vi "UHR-Fleezers Control (host) - Avogadro v2.vi"() -> ()   [LabVIEW 2014] (continued)
            n469 = local write "Stage Control Serial Error"(w819) -> ()
            n470 = Unbundle(w816) -> (w823:dbl, w825:dbl, w821:dbl)
            n471 = Add(x=w825, y="Y change (mm)") -> (x+y=w822:dbl)
            n472 = Bundle(w823, w822, w821) -> (w820:cluster{dbl, dbl, dbl})  [unwired: 1 in]
          }
          frame #1 {
            # "move to new position and start saving"
            n473 = local write "Stage Moving"(TRUE ("Stage Moving")) -> ()
            n474 = local write "Start Saving"(TRUE ("Start Saving")) -> ()
            n475 = call "Set Stage Position.vi"("Position"=w833, "error in"=w832, "VISA resource name in"=w831) -> ("error out"=w829:errorcluster, "VISA resource name out"=w830:refnum<visa-resource-name>)  [unwired: 1 out]
          }
          frame #2 {
            # "go back to start"
            n476 = call "Set Stage Position.vi"("Position"=w835, "error in"=w836, "VISA resource name in"=w837) -> ()  [unwired: 3 out]
          }
          frame #3 {
            # "stop saving"
            n477 = local write "Stop Saving"(TRUE ("Stop Saving")) -> ()
            n478 = local write "Stage Moving"(FALSE ("Stage Moving")) -> ()
          }
        }
      }
      event "Move to Position 1", "Move to Position 2", "Move to Position 3", "Move to Position 4", "Move to Position 5", "Lower Ch. Cap.", "Move to Position 6": Value Change {
        w840 = FALSE
        n479 = event-data() -> ()  [unwired: 1 in, 5 out]
        n480 = Or(x="Move to Position 5", y="Lower Ch. Cap.") -> (x .or. y?=w845:bool)
        n481 = Build Array("Move to Position 1", "Move to Position 2", "Move to Position 3", "Move to Position 4", w845, "Move to Position 6") -> (w848:bool[])
        n482 = local write "Move to Position 1"(w840) -> ()
        n483 = local write "Move to Position 2"(w840) -> ()
        n484 = local write "Move to Position 3"(w840) -> ()
        n485 = local write "Move to Position 4"(w840) -> ()
        n486 = local write "Move to Position 5"(w840) -> ()
        n487 = local write "Move to Position 6"(w840) -> ()
        n488 = Boolean Array To Number(Boolean array=w848) -> (number=w847:u32)
        n489 = Logarithm Base 2(1:w847) -> (0:w846:dbl)
        n490 = flat-sequence {
          tunnel: w846 -> [w857]
          tunnel: w843 -> [w855]
          tunnel: w842 -> [w854]
          frame #0 {
            n491 = local read "Saved Stage Positions"() -> (w865:dbl[][])
            n492 = Array Subset(array=w865, index (row)=w857, length (row)=1 ("length"), index (col)=1 ("index"), length (col)=3 ("length")) -> (w862:dbl[][])
            n493 = Reshape Array(w862, 3 ("dimension size")) -> (w860:dbl[])
            n494 = Array To Cluster(array=w860) -> (cluster=w859:cluster{"[0]":dbl, "[1]":dbl, "[2]":dbl})
            n495 = call "Set Stage Position.vi"("Position"=w859, "error in"=w854, "VISA resource name in"=w855) -> ("error out"=w858:errorcluster)  [unwired: 2 out]
            n496 = local write "Stage Moving"(TRUE ("Stage Moving")) -> ()
            n497 = local write "Stage Control Serial Error"(w858) -> ()
          }
          frame #1 {
            n498 = local write "Stage Moving"(FALSE ("Stage Moving")) -> ()
            n499 = call <vilib>:"Beep.vi"() -> ()  [unwired: 3 in, 9 out]
          }
        }
      }
      event "Force FB Data\nScript": Value Change {
        n500 = event-data() -> ()  [unwired: 1 in, 5 out]
        n501 = flat-sequence {
          tunnel: w873 -> [w877]
          tunnel: w874 -> [w878]
          tunnel: [w878] -> w869
          tunnel: [w877] -> w868
          tunnel: w869 -> [w881]
          tunnel: w868 -> [w880]
          tunnel: ["Trap Trig Fl."] -> w870
          tunnel: [w906] -> w871
          tunnel: w870 -> [w906]
          tunnel: [w910] -> w872
          tunnel: w871 -> [w910]
          tunnel: w872 -> [w912]
          frame #0 {
            n502 = property on="Trap Delta (MHz)" class="DigNum (strict)"("Val(Sgnl)"="Trap Delta Before Moving") -> ()  [unwired: 2 in, 2 out]
          }
          frame #1 {
            n503 = local read "Saved Stage Positions"() -> (w883:dbl[][])
            n504 = property on="Trap Pos. FB Offset Factor" class="DigNum (strict)"("Val(Sgnl)"=i64 0 ("Value (Signaling)")) -> ()  [unwired: 2 in, 2 out]
            n505 = local write "FB Trap Pos Offset"(0.0 ("FB Trap Pos Offset")) -> ()
            n506 = local write "Stage Moving"(TRUE ("Stage Moving")) -> ()
            n507 = call "move to saved stage position.vi"("error in"=w880, "Stage VISA resource name in"=w881, "Position"="Stage Position To Establish FB", "Saved Stage Positions"=w883) -> ("error out"=w879:errorcluster)  [unwired: 1 out]
            n508 = local write "Stage Control Serial Error"(w879) -> ()
          }
          frame #2 {
            n509 = call <vilib>:"Beep.vi"() -> ()  [unwired: 3 in, 9 out]
            n510 = Multiply(x="Wait (s)", y=u32 1000 ("milliseconds to wait")) -> (x*y=w890:u32)
            n511 = property on="Trap Delta (MHz)" class="DigNum (strict)"("Val(Sgnl)"="Starting \nTrap Delta (MHz)") -> ()  [unwired: 2 in, 2 out]
            n512 = local write "Stage Moving"(FALSE ("Stage Moving")) -> ()
            n513 = Wait (ms)(milliseconds to wait=w890) -> ()  [unwired: 1 out]
            n514 = property on="Tab Control 2" class="TabCtl (strict)"("Val(Sgnl)"=T15."Feedback on Trap Position" ("Value (Signaling)")) -> ()  [unwired: 2 in, 2 out]
            n515 = property on="Tab Control" class="TabCtl (strict)"("Val(Sgnl)"=T47."Trap Control (RF)" ("Value (Signaling)")) -> ()  [unwired: 2 in, 2 out]
          }
          frame #3 {
            n516 = property on="Set Reading to\nSetpoint" class="Bool (strict)"("Val(Sgnl)"=TRUE ("Value (Signaling)")) -> ()  [unwired: 2 in, 2 out]
            n517 = Wait (ms)(milliseconds to wait=u32 500) -> ()  [unwired: 1 out]
          }
          frame #4 {
            n518 = property on="Trap Pos. FB ON" class="Bool (strict)"("Val(Sgnl)"=TRUE ("Value (Signaling)")) -> ()  [unwired: 2 in, 2 out]
            n519 = Wait (ms)(milliseconds to wait=u32 250) -> ()  [unwired: 1 out]
          }
          frame #5 {
            n520 = case shown="False" "Trap Trig Fl." {
              frame False {
                n521 = case shown="True" "Green ON after FB ON?" {
                  selector: "Green ON after FB ON?" -> [_ w905]
                  frame False {
                  }
                  frame True {
                    n522 = property on="Green Laser ON" class="Bool (strict)"("Val(Sgnl)"=w905) -> ()  [unwired: 2 in, 2 out]
                  }
                }
              }
              frame True {
              }
            }
            n523 = case shown="True" "Remove Action Offset" {
              tunnel: TRUE ("Value (Signaling)") -> [w902 w903]
              frame False {
                n524 = property on="Remove Unwinding Offset" class="Bool (strict)"("Val(Sgnl)"=w902) -> ()  [unwired: 2 in, 2 out]
              }
              frame True {
                n525 = property on="Remove Action Offset" class="Bool (strict)"("Val(Sgnl)"=w903) -> ()  [unwired: 2 in, 2 out]
              }
            }
            n526 = Wait (ms)(milliseconds to wait=u32 250) -> ()  [unwired: 1 out]
          }
          frame #6 {
            n527 = property on="Start Saving" class="Bool (strict)"("Val(Sgnl)"=TRUE ("Value (Signaling)")) -> ()  [unwired: 2 in, 2 out]
            n528 = Wait (ms)(milliseconds to wait=u32 5000) -> ()  [unwired: 1 out]
          }
          frame #7 {
            w909 = TRUE ("Value (Signaling)")
            n529 = property on="Rem fb disp offset" class="Bool (strict)"("Val(Sgnl)"=w909) -> ()  [unwired: 2 in, 2 out]
            n530 = property on="Remove Offset" class="Bool (strict)"("Val(Sgnl)"=w909) -> ()  [unwired: 2 in, 2 out]
            n531 = Wait (ms)(milliseconds to wait=u32 100) -> ()  [unwired: 1 out]
          }
          frame #8 {
            n532 = case shown="True" w912 {
              frame False {
              }
              frame True {
                n533 = local write "Trap Trig. Fl."(TRUE ("Value (Signaling)")) -> ()
              }
            }
          }
          frame #9 {
            n534 = case shown="True" "Start dipping after?" {
              frame False {
              }
              frame True {
                n535 = flat-sequence {
                  frame #0 {
                    n536 = Multiply(x="Delay before dipping (s)", y=1000.0) -> (x*y=w916:dbl)
                    n537 = Wait (ms)(milliseconds to wait=w916) -> ()  [unwired: 1 out]
                  }
                  frame #1 {
                    n538 = property on="Dip for Protein" class="Bool (strict)"("Val(Sgnl)"=TRUE ("Value (Signaling)")) -> ()  [unwired: 2 in, 2 out]
                    n539 = local write "Scripts"(T3."Dipping" ("Scripts")) -> ()
                  }
                }
              }
            }
          }
        }
      }
      event "Fixed Traps Data\nScript": Value Change {
        n540 = event-data() -> ()  [unwired: 1 in, 5 out]
        n541 = flat-sequence {
          frame #0 {
            n542 = case shown="True" "Green ON" {
              frame False {
              }
              frame True {
                n543 = property on="Green Laser ON" class="Bool (strict)"("Val(Sgnl)"=TRUE) -> ()  [unwired: 2 in, 2 out]
              }
            }
            n544 = local write "Offset (nm)"(0.0 ("Offset (nm)")) -> ()
            n545 = property on="Sample Channel\nFlow" class="Bool (strict)"("Val(Sgnl)"=FALSE ("Value (Signaling)")) -> ()  [unwired: 2 in, 2 out]
            n546 = property on="Trap Delta (MHz)" class="DigNum (strict)"("Val(Sgnl)"="Fixed Traps Trap Delta (MHz)") -> ()  [unwired: 2 in, 2 out]
          }
          frame #1 {
            n547 = Wait (ms)(milliseconds to wait=u32 1000) -> ()  [unwired: 1 out]
          }
          frame #2 {
            n548 = local write "Start Saving"(TRUE ("Start Saving")) -> ()
          }
          frame #3 {
            n549 = local read "Bead Sep. Int. Time (s)"() -> (w927:dbl)
            n550 = Multiply(x=w927, y=1000.0) -> (x*y=w929:dbl)
            n551 = Wait (ms)(milliseconds to wait=w929) -> ()  [unwired: 1 out]
          }
          frame #4 {
            n552 = property on="Remove Offset" class="Bool (strict)"("Val(Sgnl)"=TRUE ("Value (Signaling)")) -> ()  [unwired: 2 in, 2 out]
          }
          frame #5 {
            n553 = property on="Dip for Protein" class="Bool (strict)"("Val(Sgnl)"="Start dipping after?") -> ()  [unwired: 2 in, 2 out]
          }
        }
      }
      event "Experiment position", "Get Bead 1", "Get bead 2", "Get bead 3": Value Change {
        w932 = FALSE
        n554 = event-data() -> ()  [unwired: 1 in, 6 out]
        n555 = Build Array("Get Bead 1", "Get bead 2", "Get bead 3", "Experiment position") -> (w937:bool[])
        n556 = Boolean Array To Number(Boolean array=w937) -> (number=w936:u32)
        n557 = local write "Get bead 3"(w932) -> ()
        n558 = local write "Get Bead 1"(w932) -> ()
        n559 = local write "Experiment position"(w932) -> ()
        n560 = local write "Get bead 2"(w932) -> ()
        n561 = Logarithm Base 2(1:w936) -> (0:w935:dbl)
        n562 = To Unsigned Long Integer(number=w935) -> (unsigned 32bit integer=w934:u32)
        n563 = case shown="3" w934 {
          frame 0, Default {
            n564 = property on="Move to Position 1" class="Bool (strict)"("Val(Sgnl)"=TRUE) -> ()  [unwired: 2 in, 2 out]
          }
          frame 1 {
            n565 = property on="Move to Position 2" class="Bool (strict)"("Val(Sgnl)"=TRUE) -> ()  [unwired: 2 in, 2 out]
          }
          frame 2 {
            n566 = property on="Move to Position 3" class="Bool (strict)"("Val(Sgnl)"=TRUE) -> ()  [unwired: 2 in, 2 out]
          }
          frame 3 {
            n567 = property on="Move to Position 4" class="Bool (strict)"("Val(Sgnl)"=TRUE) -> ()  [unwired: 2 in, 2 out]
          }
        }
      }
      event "Take Stepping Data": Value Change {
        n568 = event-data() -> ()  [unwired: 1 in, 5 out]
        n569 = local read "Save ave N"() -> (w953:dbl)
        n570 = flat-sequence {
          tunnel: w953 -> [w955]
          tunnel: [w955] -> w948
          tunnel: [w957] -> w949
          tunnel: w948 -> [w957]
          tunnel: [w959] -> w950
          tunnel: w949 -> [w959]
          tunnel: [w962] -> w951
          tunnel: w950 -> [w962]
          tunnel: [w964] -> w952
          tunnel: w951 -> [w964]
          tunnel: [w966] -> w946
          tunnel: w952 -> [w966]
          tunnel: w946 -> [w969]
          tunnel: [w969] -> w945
          tunnel: w945 -> [w970]
          tunnel: [w970] -> w947
          tunnel: w947 -> [w976]
          frame #0 {
            n571 = property on="Save ave N" class="DigNum (strict)"("Val(Sgnl)"="Save ave factor") -> ()  [unwired: 2 in, 2 out]
          }
          frame #1 {
            n572 = Wait (ms)(milliseconds to wait=u32 100) -> ()  [unwired: 1 out]
          }
          frame #2 {
            n573 = local read "Offset 2 Start (MHz)"() -> (w961:dbl)
            n574 = property on="Saved AOD Raster Scan Parameter Sets" class="Arr (strict)"("Index Values"=u32[] [2]) -> ()  [unwired: 2 in, 2 out]
            n575 = property on="Trap Delta (MHz)" class="DigNum (strict)"("Val(Sgnl)"=w961) -> ()  [unwired: 2 in, 2 out]
          }
          frame #3 {
            n576 = property on="Load parameters" class="Bool (strict)"("Val(Sgnl)"=TRUE ("Value (Signaling)")) -> ()  [unwired: 2 in, 2 out]
          }
          frame #4 {
            n577 = Wait (ms)(milliseconds to wait=u32 100) -> ()  [unwired: 1 out]
          }
          frame #5 {
            n578 = property on="Trap Raster Scan" class="Bool (strict)"("Val(Sgnl)"=TRUE ("Value (Signaling)")) -> ()  [unwired: 2 in, 2 out]
          }
          frame #6 {
            n579 = Wait (ms)(milliseconds to wait=u32 1000) -> ()  [unwired: 1 out]
          }
          frame #7 {
            n580 = while {
              stop <- w973 stop-if-true
              n581 = local read "Raster Scanning..."() -> (w975:bool)
              n582 = local read "Saving..."() -> (w974:bool)
              n583 = Not(x=w974) -> (.not. x?=w971:bool)
              n584 = Not(x=w975) -> (.not. x?=w972:bool)
              n585 = And(x=w972, y=w971) -> (x .and. y?=w973:bool)
            }
          }
          frame #8 {
            n586 = property on="Save ave N" class="DigNum (strict)"("Val(Sgnl)"=w976) -> ()  [unwired: 2 in, 2 out]
          }
        }
      }
      event "Step Size (nm)": Value Change {
        n587 = event-data() -> ()  [unwired: 1 in, 5 out]
        n588 = flat-sequence {
          frame #0 {
            n589 = property on="Saved AOD Raster Scan Parameter Sets" class="Arr (strict)"("Index Values"=u32[] [1]) -> ()  [unwired: 2 in, 2 out]
          }
          frame #1 {
            n590 = Multiply(x="N Steps", y="Step Size (nm)") -> (x*y=w978:dbl)
            n591 = property on="Scan Speed AOD (nm/s) 2" class="DigNum (strict)"("Value"="Step Size (nm)") -> ()  [unwired: 2 in, 2 out]
            n592 = property on="Step Size AOD (nm) 2" class="DigNum (strict)"("Value"="Step Size (nm)") -> ()  [unwired: 2 in, 2 out]
            n593 = property on="Scan Range AOD (nm) 2" class="DigNum (strict)"("Value"=w978) -> ()  [unwired: 2 in, 2 out]
          }
        }
      }
      event "Take Detection Laser\nImage": Value Change {
        n594 = event-data() -> ()  [unwired: 1 in, 5 out]
        n595 = local read "RF BD 2 to green AOM"() -> (w1007:bool)
        n596 = flat-sequence {
          tunnel: [w1039] -> w1025
          tunnel: [w1038] -> w1018
          tunnel: [w1037] -> w1010
          tunnel: [w1036] -> w1008
          tunnel: w1007 -> [w1036]
          tunnel: [w1035] -> w1000
          tunnel: [w1034] -> w988
          tunnel: [w1033] -> w981
          tunnel: [w1046] -> w1026
          tunnel: w1025 -> [w1046]
          tunnel: [w1045] -> w1019
          tunnel: w1018 -> [w1045]
          tunnel: [w1044] -> w1011
          tunnel: w1010 -> [w1044]
          tunnel: [w1043] -> w1009
          tunnel: w1008 -> [w1043]
          tunnel: [w1042] -> w1001
          tunnel: w1000 -> [w1042]
          tunnel: [w1041] -> w989
          tunnel: w988 -> [w1041]
          tunnel: [w1040] -> w982
          tunnel: w981 -> [w1040]
          tunnel: [w1054] -> w1027
          tunnel: w1026 -> [w1054]
          tunnel: [w1053] -> w1020
          tunnel: w1019 -> [w1053]
          tunnel: [w1052] -> w1012
          tunnel: w1011 -> [w1052]
          tunnel: w1009 -> [w1051]
          tunnel: [w1051] -> w1002
          tunnel: w1001 -> [w1050]
          tunnel: [w1050] -> w995
          tunnel: [w1049] -> w990
          tunnel: w989 -> [w1049]
          tunnel: [w1048] -> w983
          tunnel: w982 -> [w1048]
          tunnel: [w1065] -> w1028
          tunnel: w1027 -> [w1065]
          tunnel: [w1064] -> w1021
          tunnel: w1020 -> [w1064]
          tunnel: [w1063] -> w1013
          tunnel: w1012 -> [w1063]
          tunnel: [w1062] -> w1003
          tunnel: w1002 -> [w1062]
          tunnel: [w1061] -> w996
          tunnel: w995 -> [w1061]
          tunnel: [w1060] -> w991
          tunnel: w990 -> [w1060]
          tunnel: [w1059] -> w984
          tunnel: w983 -> [w1059]
          tunnel: [w1073] -> w1029
          tunnel: w1028 -> [w1073]
          tunnel: [w1072] -> w1022
          tunnel: w1021 -> [w1072]
          tunnel: [w1071] -> w1014
          tunnel: w1013 -> [w1071]
          tunnel: [w1070] -> w1004
          tunnel: w1003 -> [w1070]
          tunnel: [w1069] -> w997
          tunnel: w996 -> [w1069]
          tunnel: [w1068] -> w992
          tunnel: w991 -> [w1068]
          tunnel: [w1067] -> w985
          tunnel: w984 -> [w1067]
          tunnel: [w1081] -> w1030
          tunnel: w1029 -> [w1081]
          tunnel: [w1080] -> w1023
          tunnel: w1022 -> [w1080]
          tunnel: [w1079] -> w1015
          tunnel: w1014 -> [w1079]
          tunnel: [w1078] -> w1005
          tunnel: w1004 -> [w1078]
          tunnel: [w1077] -> w998
          tunnel: w997 -> [w1077]
          tunnel: [w1076] -> w993
          tunnel: w992 -> [w1076]
          tunnel: [w1075] -> w986
          tunnel: w985 -> [w1075]
          tunnel: [w1089] -> w1031
          tunnel: w1030 -> [w1089]
          tunnel: [w1088] -> w1024
          tunnel: w1023 -> [w1088]
          tunnel: [w1087] -> w1016
          tunnel: w1015 -> [w1087]
          tunnel: [w1086] -> w1006
          tunnel: w1005 -> [w1086]
          tunnel: [w1085] -> w999
          tunnel: w998 -> [w1085]
          tunnel: [w1084] -> w994
          tunnel: w993 -> [w1084]
          tunnel: [w1083] -> w987
          tunnel: w986 -> [w1083]
          tunnel: w1031 -> [w1099]
          tunnel: w1024 -> [w1098]
          tunnel: [w1096] -> w1017
          tunnel: w1016 -> [w1096]
          tunnel: w1006 -> [w1095]
          tunnel: w999 -> [w1094]
          tunnel: w994 -> [w1093]
          tunnel: w987 -> [w1092]
          tunnel: w1017 -> [w1103]
          frame #0 {
            n597 = local read "BD 2 Amplitude 2 (%)"() -> (w1034:dbl)
            n598 = local read "BD 2 Amplitude 1 (%)"() -> (w1035:dbl)
            n599 = local read "BD 2 Amplitude 3 (%)"() -> (w1033:dbl)
            n600 = local read "Laser interlacing mode"() -> (w1038:enum32{"Laser ON", "Laser OFF", "Interlace"})
            n601 = local read "Green FB On/Off"() -> (w1037:bool)
            n602 = local read "Green Laser ON"() -> (w1039:bool)
          }
          frame #1 {
            n603 = property on="Green FB On/Off" class="Bool (strict)"("Val(Sgnl)"=FALSE ("Value (Signaling)")) -> ()  [unwired: 2 in, 2 out]
          }
          frame #2 {
            n604 = case shown="True" w1051 {
              frame False {
              }
              frame True {
                w1058 = 30.0
                n605 = property on="BD 2 Amplitude 1 (%)" class="DigNum (strict)"("Val(Sgnl)"=w1058) -> ()  [unwired: 2 in, 2 out]
                n606 = property on="BD 2 Amplitude 2 (%)" class="DigNum (strict)"("Val(Sgnl)"=w1058) -> ()  [unwired: 2 in, 2 out]
                n607 = property on="BD 2 Amplitude 3 (%)" class="DigNum (strict)"("Val(Sgnl)"=w1058) -> ()  [unwired: 2 in, 2 out]
              }
            }
            n608 = property on="Green Laser ON" class="Bool (strict)"("Val(Sgnl)"=TRUE ("Value (Signaling)")) -> ()  [unwired: 2 in, 2 out]
            n609 = property on="Flip Green Filter" class="Bool (strict)"("Val(Sgnl)"=TRUE ("Value (Signaling)")) -> ()  [unwired: 2 in, 2 out]
            n610 = property on="Laser interlacing mode" class="RadioBtnsControl (strict)"("Val(Sgnl)"=enum32{"Laser ON", "Laser OFF", "Interlace"}."Laser ON" ("Value (Signaling)")) -> ()  [unwired: 2 in, 2 out]
          }
          frame #3 {
            n611 = Wait (ms)(milliseconds to wait=u32 500) -> ()  [unwired: 1 out]
          }
          frame #4 {
            n612 = property on="Confocal Image" class="Bool (strict)"("Val(Sgnl)"=TRUE ("Value (Signaling)")) -> ()  [unwired: 2 in, 2 out]
          }
          frame #5 {
            n613 = Wait (ms)(milliseconds to wait=u32 2000) -> ()  [unwired: 1 out]
          }
          frame #6 {
            n614 = while {
              stop <- w1090 stop-if-true
              n615 = local read "Saving..."() -> (w1091:bool)
              n616 = Not(x=w1091) -> (.not. x?=w1090:bool)
            }
          }
          frame #7 {
            n617 = case shown="True" w1095 {
              tunnel: w1094 -> [_ w1102]
              tunnel: w1093 -> [_ w1101]
              tunnel: w1092 -> [_ w1100]
              frame False {
              }
              frame True {
                n618 = property on="BD 2 Amplitude 1 (%)" class="DigNum (strict)"("Val(Sgnl)"=w1102) -> ()  [unwired: 2 in, 2 out]
                n619 = property on="BD 2 Amplitude 2 (%)" class="DigNum (strict)"("Val(Sgnl)"=w1101) -> ()  [unwired: 2 in, 2 out]
                n620 = property on="BD 2 Amplitude 3 (%)" class="DigNum (strict)"("Val(Sgnl)"=w1100) -> ()  [unwired: 2 in, 2 out]
              }
            }
            n621 = property on="Flip Green Filter" class="Bool (strict)"("Val(Sgnl)"=TRUE ("Value (Signaling)")) -> ()  [unwired: 2 in, 2 out]
            n622 = property on="Green Laser ON" class="Bool (strict)"("Val(Sgnl)"=w1099) -> ()  [unwired: 2 in, 2 out]
            n623 = property on="Laser interlacing mode" class="RadioBtnsControl (strict)"("Val(Sgnl)"=w1098) -> ()  [unwired: 2 in, 2 out]
          }
          frame #8 {
            n624 = property on="Green FB On/Off" class="Bool (strict)"("Val(Sgnl)"=w1103) -> ()  [unwired: 2 in, 2 out]
          }
        }
      }
      event "Move in a Circle": Value Change {
        w1105 = dbl[] []
        # "converting distance (d) to angle (a)\na=arcsin(d/2r)"
        # "radius"
        # "radius"
        # "T1 Y"
        # "T1 X"
        n625 = event-data() -> ()  [unwired: 1 in, 5 out]
        n626 = local read "BD 1 Frequency 1 (MHz)"() -> (w1113:dbl)
        n627 = local read "BD 2 Frequency 1 (MHz)"() -> (w1112:dbl)
        n628 = local read "BD 1 Frequency 2 (MHz)"() -> (w1111:dbl)
        n629 = local read "BD 2 Frequency 2 (MHz)"() -> (w1110:dbl)
        n630 = Subtract(x=w1112, y="Center Y Frequency (MHz)") -> (x-y=w1117:dbl)
        n631 = Absolute Value(x=w1117) -> (abs(x)=w1108:dbl)
        n632 = flat-sequence {
          tunnel: w1108 -> [w1120]
          tunnel: [w1120] -> w1107
          frame #0 {
            n633 = local write "Radius (MHz)"(w1120) -> ()
          }
        }
        n634 = node-c288("Time step (ms)") -> (w1119:T42)  [unwired: 3 in]
        n635 = timed-loop {
          timing: w1119 -> [_]
          timing-out: [_] -> w1118
          tunnel: w1113 -> [w1211]
          tunnel: w1112 -> [_]
          tunnel: w1111 -> [w1215]
          tunnel: w1110 -> [_]
          tunnel: "Center Y Frequency (MHz)" -> [w1204]
          shift-right: [w1165] -> _
          shift-left: w1105 -> [w1172]
          shift-right: [w1163] -> _
          shift-left: w1105 -> [w1171]
          shift-right: [w1156] -> _
          shift-left: w1105 -> [w1169]
          shift-right: [w1154] -> _
          shift-left: w1105 -> [w1168]
          tunnel: "Move in a Circle" -> [_]
          tunnel: ["Back to start on finish?"] -> w1109
          tunnel: w1107 -> [_]
          tunnel: w1106 -> [w1186]
          tunnel: w1105 -> [w1167]
          shift-right: [w1138] -> _
          shift-left: 0.0 -> [w1136]
          i -> [w1145]
          stop <- w1209 stop-if-true
          w1153 = 0 ("index")
          w1174 = 1 ("dimension size")
          # "Keep phase within\n2pi so errors don't \nbuild"
          # "Accumulated\nphase"
          # "Current phase"
          # "Trap 2"
          # "Trap 1"
          # "ignore if N = 0"
          # "r"
          # "r"
          # "r"
          # "r"
          # "\"omega*t\""
          # "Trap 2"
          # "Trap separation (radians)"
          # "Trap 1"
          # "Offset (starts\n at bottom of\n the circle)"
          # "omega"
          n636 = node-c288() -> (w1222:i64)  [unwired: 1 in]
          n637 = Divide(x=w1222, y=1000) -> (x/y=w1141:dbl)
          n638 = Divide(x="2D Motion Trap Separation (MHz)", y="Radius (MHz)") -> (x/y=w1196:dbl)
          n639 = Negate(x=w1141) -> (-x=w1140:dbl)
          n640 = Divide(x="Trap 2 phase shift (deg)", y=360.0) -> (x/y=w1187:dbl)
          n641 = Inverse Sine(1:w1196) -> (0:w1132:dbl)
          n642 = Multiply(x=6.283185307179586, y=w1187) -> (x*y=w1133:dbl)
          n643 = Multiply(x=6.283185307179586, y="2D Motion Frequency (Hz)") -> (x*y=w1144:dbl)
          n644 = Select(t=w1141, s="Counterclockwise/Clockwise", f=w1140) -> (s? t:f=w1143:dbl)
          n645 = Multiply(x=w1144, y=w1143) -> (x*y=w1134:dbl)
          n646 = Select(t=w1132, s="Trap shift\nmethod", f=w1133) -> (s? t:f=w1131:dbl)
          n647 = Add(x=w1134, y=w1136) -> (x+y=w1137:dbl)
          n648 = Add(x=w1137, y=w1131) -> (x+y=w1193:dbl)
          n649 = Add(x=w1137, y=1.5707963267948966) -> (x+y=w1142:dbl)
          n650 = Add(x=w1193, y=1.5707963267948966) -> (x+y=w1206:dbl)
          n651 = Cosine(x=w1142) -> (cos(x)=w1220:dbl)
          n652 = Sine(x=w1142) -> (sin(x)=w1219:dbl)
          n653 = Multiply(x=w1220, y="Radius (MHz)") -> (x*y=w1213:dbl)
          n654 = Cosine(x=w1206) -> (cos(x)=w1218:dbl)
          n655 = Sine(x=w1206) -> (sin(x)=w1217:dbl)
          n656 = Multiply(x=w1219, y="Radius (MHz)") -> (x*y=w1212:dbl)
          n657 = Multiply(x=w1218, y="Radius (MHz)") -> (x*y=w1216:dbl)
          n658 = Multiply(x=w1217, y="Radius (MHz)") -> (x*y=w1214:dbl)
          n659 = Add(x=w1213, y=w1211) -> (x+y=w1162:dbl)
          n660 = Add(x=w1212, y=w1204) -> (x+y=w1160:dbl)
          n661 = Greater Or Equal?(x=w1145, y="N steps then stop") -> (x >= y?=w1203:bool)
          n662 = Add(x=w1216, y=w1215) -> (x+y=w1151:dbl)
          n663 = Add(x=w1214, y=w1204) -> (x+y=w1149:dbl)
          n664 = Not Equal To 0?(x="N steps then stop") -> (x != 0?=w1199:bool)
          n665 = And(x=w1203, y=w1199) -> (x .and. y?=w1200:bool)
          n666 = local read "Trap 1 sum mean"() -> (w1183:dbl)
          n667 = local read "Stop All"() -> (w1208:bool)
          n668 = local write "BD 1 Frequency 1 (MHz)"(w1162) -> ()
          n669 = local write "BD 2 Frequency 1 (MHz)"(w1160) -> ()
          n670 = local write "BD 1 Frequency 2 (MHz)"(w1151) -> ()
          n671 = local write "BD 2 Frequency 2 (MHz)"(w1149) -> ()
          n672 = Select(t=w1145, s="test", f=w1183) -> (s? t:f=→"Waveform Chart":dbl)
          n673 = Compound Arithmetic op=OR(w1208, "Stop Moving", w1200) -> (w1209:bool)
          n674 = local read "BD 1 Frequency 3 (MHz)"() -> (w1192:dbl)
          n675 = local read "BD 2 Frequency 3 (MHz)"() -> (w1191:dbl)
          n676 = Select(t=w1167, s="Reset graph", f=w1168) -> (s? t:f=w1148:dbl[])
          n677 = Select(t=w1167, s="Reset graph", f=w1169) -> (s? t:f=w1150:dbl[])
          n678 = Select(t=w1167, s="Reset graph", f=w1171) -> (s? t:f=w1159:dbl[])
          n679 = Select(t=w1167, s="Reset graph", f=w1172) -> (s? t:f=w1161:dbl[])
          n680 = Initialize Array(w1149, w1174) -> (w1175:dbl[])
          n681 = Initialize Array(w1160, w1174) -> (w1178:dbl[])
          n682 = Initialize Array(w1151, w1174) -> (w1176:dbl[])
          n683 = Initialize Array(w1162, w1174) -> (w1179:dbl[])
          n684 = local read "Y RF Frequency Limits (MHz)"() -> (w1189:T26)
          n685 = local read "X RF Frequency Limits (MHz)"() -> (w1190:T26)
          n686 = call "set RF board frequency - interlace.vi"("Board 2 Frequency Limits"=w1189, "Board 1 Frequency Limits"=w1190, "FPGA VI Reference In"=w1186, "Board 2 Frequency 3 (MHz)"=w1191, "Board 1 Frequency 3 (MHz)"=w1192, "Board 2 Frequency 2 (MHz)"=w1149, "Board 2 Frequency 1 (MHz)"=w1160, "Board 1 Frequency 2 (MHz)"=w1151, "Board 1 Frequency 1  (MHz)"=w1162) -> ()  [unwired: 1 in, 2 out]
          n687 = Bundle(w1176, w1175) -> (w1147:cluster{dbl[], dbl[]})  [unwired: 1 in]
          n688 = Bundle(w1179, w1178) -> (w1177:cluster{dbl[], dbl[]})  [unwired: 1 in]
          n689 = Build Array (concatenate)(w1162, w1161) -> (w1166:dbl[])
          n690 = Build Array (concatenate)(w1160, w1159) -> (w1164:dbl[])
          n691 = Build Array (concatenate)(w1151, w1150) -> (w1157:dbl[])
          n692 = Build Array (concatenate)(w1149, w1148) -> (w1155:dbl[])
          n693 = Bundle(w1166, w1164) -> (w1146:cluster{dbl[], dbl[]})  [unwired: 1 in]
          n694 = Bundle(w1157, w1155) -> (w1173:cluster{dbl[], dbl[]})  [unwired: 1 in]
          n695 = Build Array(w1177, w1147, w1146, w1173) -> (→"Trap trajectories":cluster{dbl[], dbl[]}[])
          n696 = case "To pause the process" shown="True" "Pause rotation" {
            frame False {
            }
            frame True {
              n697 = while {
                stop <- w1225 stop-if-true
                n698 = local read "Pause rotation"() -> (w1226:bool)
                n699 = Wait (ms)(milliseconds to wait=u32 10) -> ()  [unwired: 1 out]
                n700 = Not(x=w1226) -> (.not. x?=w1225:bool)
              }
            }
          }
          n701 = Decrement(x="N steps to plot") -> (x-1=w1152:i32)
          n702 = Array Subset(array=w1164, index=w1153, length=w1152) -> (w1163:dbl[])
          n703 = Array Subset(array=w1166, index=w1153, length=w1152) -> (w1165:dbl[])
          n704 = Array Subset(array=w1157, index=w1153, length=w1152) -> (w1156:dbl[])
          n705 = Array Subset(array=w1155, index=w1153, length=w1152) -> (w1154:dbl[])
          n706 = Quotient & Remainder(x=w1137, y=6.283185307179586) -> (x-y*floor(x/y)=w1138:dbl)  [unwired: 1 out]
          n707 = node-c288() -> ()  [unwired: 1 in, 1 out]
        }
        n708 = node-c288(w1118) -> ()  [unwired: 1 out]
        n709 = case shown="True" w1109 {
          tunnel: w1113 -> [_ w1124]
          tunnel: w1112 -> [_ w1123]
          tunnel: w1111 -> [_ w1122]
          tunnel: w1110 -> [_ w1121]
          frame False {
          }
          frame True {
            n710 = flat-sequence {
              tunnel: w1124 -> [w1128]
              tunnel: w1123 -> [w1127]
              tunnel: w1122 -> [w1126]
              tunnel: w1121 -> [w1125]
              frame #0 {
                n711 = local write "BD 1 Frequency 1 (MHz)"(w1128) -> ()
                n712 = local write "BD 2 Frequency 1 (MHz)"(w1127) -> ()
                n713 = local write "BD 1 Frequency 2 (MHz)"(w1126) -> ()
                n714 = local write "BD 2 Frequency 2 (MHz)"(w1125) -> ()
              }
              frame #1 {
                n715 = property on="Update all trap values" class="Bool (strict)"("Val(Sgnl)"=TRUE ("Value (Signaling)")) -> ()  [unwired: 2 in, 2 out]
              }
            }
          }
        }
      }
      event "Stop All": Value Change {
        # "Stopping blue laser before shutting off program"
        n716 = event-data() -> ()  [unwired: 1 in, 5 out]
        n717 = local read "Delay (ms)"() -> (w1236:i32)
        n718 = call "serial write macro.vi"("String"="l0", "Delay (ms)"=w1236, "VISA resource name"=w1239) -> ("read buffer"=w1234:string, "error out"=w1235:errorcluster, "VISA resource name out"=w1238:refnum<visa-resource-name>)
        n719 = local write "read blue buffer"(w1234) -> ()
        n720 = local write "Blue Error Out"(w1235) -> ()
        n721 = VISA Close(VISA resource name=w1238) -> ()  [unwired: 1 in, 1 out]
        n722 = local read "Stop All"() -> (w1240:bool)
      }
      event "Sensitivity", "Offset Current Sign", "Offset Current Value", "Offset Current", "Bias Voltage", "Bias Voltage (mV)", "Filter Type", "Lowpass 3dB Point", "Highpass 3dB Point", "Filter Reset", "Invert Signal", "Gain Mode", "Send Command": Value Change {
        w1247 = 250 ("Delay (ms)")
        n723 = event-data() -> ()  [unwired: 1 in, 5 out]
        n724 = event shown="[0] \"Sensitivity\": Value Change" {
          selector: _ -> [_ _ _ _ _ _ _ _ _ _ _ _ _]
          dyn-events: _ -> [_ _ _ _ _ _ _ _ _ _ _ _ _]
          timeout: _ -> [_ _ _ _ _ _ _ _ _ _ _ _ _]
          tunnel: [w1259 w1267 w1275 w1284 w1294 w1302 w1305 w1309 w1312 w1315 w1318 w1325 "Command"] -> w1246
          tunnel: [w1254 w1261 w1271 w1278 w1288 w1298 _ _ _ _ _ w1321 _] -> w1241
          event "Sensitivity": Value Change {
            n725 = event-data() -> ()  [unwired: 1 in, 5 out]
            n726 = property on="Sensitivity" class="CmbBox"() -> ("Value"=→"Gain":string)  [unwired: 2 in, 2 out]
            n727 = Concatenate Strings("SENS ", "Sensitivity") -> (w1259:string)
            n728 = local read "Gain"() -> (w1256:string)
            n729 = Concatenate Strings("gain set at ", w1256) -> (w1254:string)
          }
          event "Offset Current Sign": Value Change {
            n730 = event-data() -> ()  [unwired: 1 in, 4 out]
            n731 = Boolean To (0,1)(Boolean="Offset Current Sign") -> (0, 1=w1270:i16)
            n732 = Select(t="positive", s="Offset Current Sign", f="negative") -> (s? t:f=w1262:string)
            n733 = Number To Decimal String(number=w1270) -> (decimal integer string=w1269:string)  [unwired: 1 in]
            n734 = Concatenate Strings("IOSN " ("string"), w1269) -> (w1267:string)
            n735 = Concatenate Strings("offset current sign ", w1262) -> (w1261:string)
          }
          event "Offset Current Value": Value Change {
            n736 = event-data() -> ()  [unwired: 1 in, 5 out]
            n737 = property on="Offset Current Value" class="CmbBox"() -> ("Value"=→"Read offset current":string)  [unwired: 2 in, 2 out]
            n738 = local read "Read offset current"() -> (w1272:string)
            n739 = Concatenate Strings("IOLV ", "Offset Current Value") -> (w1275:string)
            n740 = Concatenate Strings("offset current value ", w1272) -> (w1271:string)
          }
          event "Offset Current": Value Change {
            n741 = event-data() -> ()  [unwired: 1 in, 5 out]
            n742 = Boolean To (0,1)(Boolean="Offset Current") -> (0, 1=w1287:i16)
            n743 = Select(t="on", s="Offset Current", f="off") -> (s? t:f=w1279:string)
            n744 = Number To Decimal String(number=w1287) -> (decimal integer string=w1286:string)  [unwired: 1 in]
            n745 = Concatenate Strings("IOON " ("string"), w1286) -> (w1284:string)
            n746 = Concatenate Strings("offset current ", w1279) -> (w1278:string)
          }
          event "Bias Voltage": Value Change {
            n747 = event-data() -> ()  [unwired: 1 in, 5 out]
            n748 = Boolean To (0,1)(Boolean="Bias Voltage") -> (0, 1=w1295:i16)
            n749 = Number To Decimal String(number=w1295) -> (decimal integer string=w1296:string)  [unwired: 1 in]
            n750 = Select(t="on", s="Bias Voltage", f="off") -> (s? t:f=w1289:string)
            n751 = Concatenate Strings("BSON " ("string"), w1296) -> (w1294:string)
            n752 = Concatenate Strings("bias voltage", w1289) -> (w1288:string)
          }
          event "Bias Voltage (mV)": Value Change {
            n753 = event-data() -> ()  [unwired: 1 in, 5 out]
            n754 = Number To Decimal String(number="Bias Voltage (mV)") -> (decimal integer string=w1304:string)  [unwired: 1 in]
            n755 = Number To Fractional String(number="Bias Voltage (mV)") -> (F-format string=w1299:string)  [unwired: 3 in]
            n756 = Concatenate Strings("BSLV " ("string"), w1304) -> (w1302:string)
            n757 = Concatenate Strings("bias voltage value ", w1299) -> (w1298:string)
          }
          event "Filter Type": Value Change {
            n758 = event-data() -> ()  [unwired: 1 in, 5 out]
            n759 = Concatenate Strings("FLTT " ("string"), "Filter Type") -> (w1305:string)
          }
          event "Lowpass 3dB Point": Value Change {
            n760 = event-data() -> ()  [unwired: 1 in, 5 out]
            n761 = Concatenate Strings("LFRQ " ("string"), "Lowpass 3dB Point") -> (w1309:string)
          }
          event "Highpass 3dB Point": Value Change {
            n762 = event-data() -> ()  [unwired: 1 in, 5 out]
            n763 = Concatenate Strings("HFRQ " ("string"), "Highpass 3dB Point") -> (w1312:string)
          }
          event "Filter Reset": Value Change {
            n764 = event-data() -> ()  [unwired: 1 in, 5 out]
            n765 = Select(t="ROLD", s="Filter Reset", f="") -> (s? t:f=w1315:string)
          }
          event "Gain Mode": Value Change {
            n766 = event-data() -> ()  [unwired: 1 in, 5 out]
            n767 = Concatenate Strings("GNMD " ("string"), "Gain Mode") -> (w1318:string)
          }
          event "Invert Signal": Value Change {
            n768 = event-data() -> ()  [unwired: 1 in, 5 out]
            n769 = Boolean To (0,1)(Boolean="Invert Signal") -> (0, 1=w1328:i16)
            n770 = Number To Decimal String(number=w1328) -> (decimal integer string=w1327:string)  [unwired: 1 in]
            n771 = Concatenate Strings("INVT " ("string"), w1327) -> (w1325:string)
            n772 = Select(t="signal inverted", s="Invert Signal", f="signal not inverted") -> (s? t:f=w1321:string)
          }
          event "Send Command": Value Change {
            n773 = event-data() -> ()  [unwired: 1 in, 5 out]
          }
        }
        "Command Sent" <- w1246
        n774 = local read "Save Event Log?"() -> (w1242:bool)
        n775 = local read "Saving..."() -> (w1243:bool)
        n776 = And(x=w1242, y=w1243) -> (x .and. y?=w1244:bool)
        n777 = case shown="True" w1244 {
          tunnel: w1241 -> [_ w1251]
          frame False {
          }
          frame True {
            n778 = local read "Time (s)"() -> (w1252:dbl)
            n779 = local read "log file ref"() -> (w1253:refnum<file>)
            n780 = call "write to event log.vi"("log file ref"=w1253, "time"=w1252, "input string"=w1251) -> ()  [unwired: 8 in]
          }
        }
        n781 = call "preamp serial write macro.vi"("String"=w1246, "Delay (ms)"=w1247, "VISA resource name"=w1250) -> ("read buffer"=→"Reply":string, "error out"=w1249:errorcluster)  [unwired: 1 out]
        n782 = call "preamp serial write macro.vi"("String"=w1246, "Delay (ms)"=w1247, "VISA resource name"=w1245) -> ()  [unwired: 3 out]
        n783 = local write "Preamp Error Out"(w1249) -> ()
      }
    }
    n784 = node-c288() -> ()  [unwired: 1 in, 1 out]
  }
  n785 = Subtract(x=w11, y="Maximum Delta\n(MHz)") -> (x-y=w9:dbl)
  n786 = Bundle By Name(cluster=T26 {"Minimum"=60.0, "Maximum"=90.0, "Increment"=1.0} ("Min Max Inc"), "Minimum"=w9, "Maximum"=w11) -> (w8:T26)
  n787 = flat-sequence "Safety limits on RF frequencies and amplitudes (for AOM protection)" {
    tunnel: [w1332] -> w22
    tunnel: [w1330] -> w24
    tunnel: [w1333] -> w25
    tunnel: [w1334] -> w23
    tunnel: w8 -> [w1332]
    tunnel: T26 {"Minimum"=0.0, "Maximum"=50.0, "Increment"=1.0} ("Data Entry Limits") -> [w1330]
    tunnel: w1 -> [w1331]
    tunnel: [w1331] -> w26
    frame #0 {
      w1334 = T26 {"Minimum"=0.0, "Maximum"=40.0, "Increment"=0.1} ("Min Max Inc")
      w1333 = T26 {"Minimum"=0.0, "Maximum"=45.0, "Increment"=1.0} ("Data Entry Limits")
      n788 = property on="BD 2 Frequency 1 (MHz)" class="DigNum (strict)"("Data Range"=w1334) -> ()  [unwired: 2 in, 2 out]
      n789 = property on="BD 2 Frequency 3 (MHz)" class="DigNum (strict)"("Data Range"=w1334) -> ()  [unwired: 2 in, 2 out]
      n790 = property on="BD 2 Frequency 2 (MHz)" class="DigNum (strict)"("Data Range"=w1334) -> ()  [unwired: 2 in, 2 out]
      n791 = property on="BD 1 Frequency 1 (MHz)" class="DigNum (strict)"("Data Range"=w1332) -> ()  [unwired: 2 in, 2 out]
      n792 = property on="BD 1 Frequency 2 (MHz)" class="DigNum (strict)"("Data Range"=w1332) -> ()  [unwired: 2 in, 2 out]
      n793 = property on="BD 1 Frequency 3 (MHz)" class="DigNum (strict)"("Data Range"=w1332) -> ()  [unwired: 2 in, 2 out]
      n794 = property on="BD 2 Amplitude 1 (%)" class="DigNum (strict)"("Data Range"=w1333) -> ()  [unwired: 2 in, 2 out]
      n795 = property on="BD 2 Amplitude 2 (%)" class="DigNum (strict)"("Data Range"=w1333) -> ()  [unwired: 2 in, 2 out]
      n796 = property on="BD 2 Amplitude 3 (%)" class="DigNum (strict)"("Data Range"=w1333) -> ()  [unwired: 2 in, 2 out]
      n797 = property on="BD 1 Amplitude 3 (%)" class="DigNum (strict)"("Data Range"=w1330) -> ()  [unwired: 2 in, 2 out]
      n798 = property on="BD 1 Amplitude 2 (%)" class="DigNum (strict)"("Data Range"=w1330) -> ()  [unwired: 2 in, 2 out]
      n799 = property on="BD 1 Amplitude 1 (%)" class="DigNum (strict)"("Data Range"=w1330) -> ()  [unwired: 2 in, 2 out]
      "X RF Frequency Limits (MHz)" <- w1332
      "X RF Amplitude Limits (%)" <- w1330
      "Y RF Amplitude Limits (%)" <- w1333
      "Y RF Frequency Limits (MHz)" <- w1334
    }
  }
  n800 = stacked-sequence "Host initialization sequence - order matters!" {
    tunnel: w26 -> [_ w1359 w1452 _ w1509 w1518 w1558 _ _ w1698]
    tunnel: [_ _ _ _ _ _ _ _ _ w1698] -> w15
    tunnel: [_ _ _ _ _ _ _ _ _ w1697] -> w28
    tunnel: w25 -> [_ _ _ _ _ _ w1585 _ _ _]
    tunnel: w24 -> [_ _ _ _ _ _ w1584 _ _ _]
    tunnel: w23 -> [_ _ _ _ _ _ w1583 _ _ _]
    tunnel: w22 -> [_ _ _ _ _ _ w1564 _ _ _]
    tunnel: [_ _ _ _ _ _ _ _ w1686 _] -> _
    tunnel: w3 -> [_ _ _ _ _ _ _ _ w1672 _]
    frame #0 {
    }
    frame #1 {
      w1391 = 10.0 ("y")
      w1392 = 32767.0 ("y")
      w1376 = 6.0  # clock mult.
      w1375 = 49152000.0  # TCXO frequ.
      # "Initialize some FPGA settings"
      n801 = local read "Not-Interlacing Set"() -> (w1431:enum32{"Set 1", "Set 2", "Set 3"})
      n802 = local write "Trap Pos FIFO Timeout"(u16 0 ("Trap Pos FIFO Timeout")) -> ()
      n803 = local read "Interlace"() -> (w1429:bool)
      n804 = local read "Desired Scan Incr (V)"() -> (w1403:dbl)
      n805 = local read "BD 1 Delay (ticks)"() -> (w1438:u8)
      n806 = local read "Number Interlace Sets"() -> (w1430:u8)
      n807 = local read "BD 2 Delay (Ticks)"() -> (w1439:u8)
      n808 = property on="AI Count (ticks)" class="DigNum (strict)"("Val(Sgnl)"="AI Count (ticks)") -> ()  [unwired: 2 in, 2 out]
      n809 = local read "AO1"() -> (w1397:dbl)
      n810 = local read "AO2"() -> (w1398:dbl)
      n811 = local read "Next trap write delay (ticks)"() -> (w1440:u8)
      n812 = local read "Number of scans (MCL)"() -> (w1407:u64)
      n813 = local read "Cycles/step (MCL)"() -> (w1406:u64)
      n814 = local read "Scan steps (MCL)"() -> (w1405:u64)
      n815 = local read "Continuous MCL Scanning"() -> (w1408:bool)
      n816 = Multiply(x=w1397, y=w1392) -> (x*y=w1395:dbl)
      n817 = Multiply(x=w1398, y=w1392) -> (x*y=w1393:dbl)
      n818 = Build Array("DIO count 1 (ticks)", "DIO count 2 (ticks)", "DIO count 3 (ticks)") -> (w1424:u16[])
      n819 = local read "Fast Scan Dir"() -> (w1409:bool)
      n820 = local read "2D or 1D Scan"() -> (w1421:bool)
      n821 = local read "N Acq Sets (Traps + Fl.)"() -> (w1417:i16)
      n822 = local read "Scan Increment (MHz)"() -> (w1380:dbl)
      n823 = Divide(x=w1395, y=w1391) -> (x/y=w1396:dbl)
      n824 = Divide(x=w1393, y=w1391) -> (x/y=w1394:dbl)
      n825 = To Unsigned Byte Integer(number=w1431) -> (unsigned 8bit integer=w1426:u8)
      n826 = Split 1D Array(array=w1424, index=w1430) -> (first subarray=w1422:u16[])  [unwired: 1 out]
      n827 = Multiply(x=w1403, y=32767.0) -> (x*y=w1401:dbl)
      n828 = To Word Integer(number=w1396) -> (16bit integer=w1342:i16)
      n829 = To Word Integer(number=w1394) -> (16bit integer=w1341:i16)
      n830 = Index Array(array=w1424, index=w1426) -> (element=w1425:u16)
      n831 = Add Array Elements(numeric array=w1422) -> (sum=w1423:u16)
      n832 = Multiply(x=w1375, y=w1376) -> (x*y=w1377:dbl)
      n833 = Divide(x=w1401, y=10.0) -> (x/y=w1402:dbl)
      n834 = Select(t=w1423, s=w1429, f=w1425) -> (s? t:f=w1432:u16)
      n835 = Not(x=w1409) -> (.not. x?=w1410:bool)
      n836 = To Word Integer(number=w1402) -> (16bit integer=w1404:i16)
      n837 = property on="2D or 1D Scan" class="Bool (strict)"("Val(Sgnl)"=w1421) -> ()  [unwired: 2 in, 2 out]
      n838 = Divide(x=40000000.0, y="AI Count (ticks)") -> (x/y=w1413:dbl)
      n839 = local write "Update Count (MCL)"(w1432) -> ()
      n840 = local write "Total Counts (ticks)"(w1432) -> ()
      n841 = Divide(x=w1413, y="FPGA Ave.") -> (x/y=w1412:dbl)
      n842 = local write "AI rate (Hz)"(w1413) -> ()
      n843 = Multiply(x=w1380, y=1000.0) -> (x*y=w1373:dbl)
      n844 = local write "Ave. Rate (Hz)"(w1412) -> ()
      n845 = Reciprocal(x=w1412) -> (1/x=w1411:dbl)
      n846 = Scale By Power Of 2(n=48, x=w1373) -> (x*2^n=w1372:dbl)
      n847 = local write "Ave. Period (s)"(w1411) -> ()
      n848 = Divide(x=w1372, y=w1377) -> (x/y=w1378:dbl)
      n849 = To Quad Integer(1:w1378) -> (0:w1381:i64)
      n850 = local read "Setpoints (V)"() -> (w1366:cluster{"Set 1":dbl, "Set 2":dbl})
      n851 = local read "# Samples/channel"() -> (w1388:u32)
      n852 = local read "Feedback On/Off"() -> (w1363:cluster{"Set 1":bool, "Set 2":bool})
      n853 = local read "T3 Y (V)"() -> (w1346:dbl)
      n854 = local read "T3 X (V)"() -> (w1345:dbl)
      n855 = local read "Trap intensity output range"() -> (w1356:cluster{"Normal High":i16, "Normal Low":i16})
      n856 = local read "All FB On/Off"() -> (w1362:bool)
      n857 = local read "Number of F/B Scans (AOD)"() -> (w1387:u16)
      n858 = local read "Trap Intensity PID Gains"() -> (w1355:T18)
      n859 = local read "Cycles/step (AOD)"() -> (w1383:u64)
      n860 = local read "Scan steps (AOD)"() -> (w1382:u64)
      n861 = Multiply(x=w1382, y=w1383) -> (x*y=w1384:u64)
      n862 = Multiply(x=w1384, y=u64 2) -> (x*y=w1386:u64)
      n863 = Multiply(x=w1386, y=w1387) -> (x*y=w1389:u64)
      n864 = Multiply(x=3276.7, y=w1366) -> (x*y=w1367:cluster{"Set 1":dbl, "Set 2":dbl})
      n865 = local read "Scan BD"() -> (w1371:bool)
      n866 = Multiply(x=w1346, y=32767.0) -> (x*y=w1352:dbl)
      n867 = And(x=w1363, y=w1362) -> (x .and. y?=w1364:cluster{"Set 1":bool, "Set 2":bool})
      n868 = To Word Integer(number=w1367) -> (16bit integer=w1368:cluster{"Set 1":i16, "Set 2":i16})
      n869 = Multiply(x=w1345, y=32767.0) -> (x*y=w1349:dbl)
      n870 = local read "Sets to FIFO (Traps)"() -> (w1434:T25)
      n871 = Divide(x=w1389, y=w1388) -> (x/y=w1390:dbl)
      n872 = Unbundle By Name(w1364) -> ("Set 1"=w1360:bool, "Set 2"=w1361:bool)
      n873 = Unbundle By Name(w1368) -> ("Set 1"=w1369:i16, "Set 2"=w1370:i16)
      n874 = Divide(x=w1352, y=10.0) -> (x/y=w1353:dbl)
      n875 = Divide(x=w1349, y=10.0) -> (x/y=w1348:dbl)
      n876 = To Unsigned Word Integer(number=w1353) -> (unsigned 16bit integer=w1344:u16)
      n877 = To Unsigned Word Integer(number=w1348) -> (unsigned 16bit integer=w1343:u16)
      n878 = local read "FPGA error out"() -> (w1358:errorcluster)
      n879 = local write "Data points/scan (f/b)"(w1386) -> ()
      n880 = local write "Data points/scans"(w1389) -> ()
      n881 = local write "N sets should be saved"(w1390) -> ()
      n882 = Unbundle By Name(w1434) -> ("Set 1"=w1435:bool, "Set 2"=w1436:bool, "Set 3"=w1437:bool)
      n883 = xnode "Read/Write Control"("FPGA VI Reference In"=w1359, "error in"=w1358, "ai count"="AI Count (ticks)", "Interlace ON/OFF"=w1429, "Number Interlace Cycles"=w1430, "Set 1"=w1435, "Set 2"=w1436, "Set 3"=w1437, "FB On/Off Set 1"=w1360, "FB On/Off Set 2"=w1361, "Interlace Off Parameters"=w1431, "FB Setpoint Set 1"=w1369, "FB Setpoint Set 2"=w1370, "Piezo Trap Y (AO4)"=w1344, "Piezo Trap X (AO5)"=w1343, "FB Gains"=w1355, "FB output range"=w1356, "Cycles per step"=w1383, "Scan BD"=w1371, "Number of scans"=w1387, "Scan steps"=w1382, "Scan freq.  increment"=w1381, "AO1 (Y)"=w1342, "AO2 (X)"=w1341, "Scan freq.  increment (MCL)"=w1404, "Scan steps (MCL)"=w1405, "Cycles per step (MCL)"=w1406, "Number of scans (MCL)"=w1407, "MCL count"=w1432, "Cont. Scan (MCL)"=w1408, "MCL Scan Axis"=w1410, "1D or 2D Scan?"=w1421, "N of AI1 Int Acq Sets"=w1417, "Amp switch delay"="RF amplitude switch delay", "Swap F1 and F2"="Swap F1 and F2", "APD to FIFO"=FALSE, "DIO count 1 (ticks)"="DIO count 1 (ticks)", "DIO count 2 (ticks)"="DIO count 2 (ticks)", "DIO count 3 (ticks)"="DIO count 3 (ticks)", "BD 1 Delay (ticks)"=w1438, "BD 2 Delay (Ticks)"=w1439, "Next trap write delay (ticks)"=w1440, "Phase offset method"="Phase offset method", "Phase Trap 1"="Phase Increment Trap 1", "Phase Trap 2"="Phase Increment Trap 2", "RF phase reset before cycles"="RF phase reset before cycles", "RF synth bd controls green"="RF BD 2 to green AOM") -> ("error out"=w1357:errorcluster)  [unwired: 1 out]
      n884 = local write "FPGA error out"(w1357) -> ()
    }
    frame #2 {
      # "Initialize some more FPGA settings"
      n885 = local read "Trap Pos FB Monitor\nT1 or T2"() -> (w1463:bool)
      n886 = local read "Trap Pos FB Negate Action"() -> (w1464:bool)
      n887 = local read "Trap Pos. FB Offset Factor"() -> (w1465:i64)
      n888 = local read "Trap Pos. FB Mult Factor"() -> (w1466:i64)
      n889 = local read "Trap Pos. AI1 X Pre-scale"() -> (w1468:u16)
      n890 = local read "Trap Pos FB Int Count"() -> (w1470:u16)
      n891 = local read "Green Laser ON"() -> (w1442:bool)
      n892 = local read "Neg. TTrig FPGA"() -> (w1471:bool)
      n893 = local read "Trap Pos. FB Range"() -> (w1447:T22)
      n894 = local read "Trap Pos. FB Gains"() -> (w1448:T21)
      n895 = local read "Dynamic Force FB (ronen)"() -> (w1449:bool)
      n896 = Multiply(x="Green Intensity % (FB OFF)", y=655.35) -> (x*y=w1457:dbl)
      n897 = Multiply(x="Red FB Setpoint (mV)", y=3.2767) -> (x*y=w1479:dbl)
      n898 = Multiply(x="Red Intensity % (FB OFF)", y=655.35) -> (x*y=w1483:dbl)
      n899 = Unbundle By Name("Red FB Gains") -> ("proportional gain (Kc)"=w1488:i16, "integral gain (Kc*Ts/Ti)"=w1489:i16, "derivative gain (Kc*Td/Ts)"=w1490:i16)
      n900 = Multiply(x="Green FB Setpoint (mV)", y=3.2767) -> (x*y=w1460:dbl)
      n901 = To Unsigned Word Integer(number=w1457) -> (unsigned 16bit integer=w1459:u16)
      n902 = To Unsigned Word Integer(number=w1483) -> (unsigned 16bit integer=w1486:u16)
      n903 = To Word Integer(number=w1479) -> (16bit integer=w1482:i16)
      n904 = local read "Differential FB?"() -> (w1473:bool)
      n905 = To Word Integer(number=w1460) -> (16bit integer=w1462:i16)
      n906 = local read "Laser interlacing mode"() -> (w1445:enum32{"Laser ON", "Laser OFF", "Interlace"})
      n907 = local read "Invert laser interlacing"() -> (w1446:bool)
      n908 = Unbundle By Name("Green FB Gains") -> ("proportional gain (Kc)"=w1476:i16, "integral gain (Kc*Ts/Ti)"=w1477:i16, "derivative gain (Kc*Td/Ts)"=w1478:i16)
      n909 = Select(t=w1445, s=w1442, f=enum32{"Laser ON", "Laser OFF", "Interlace"}."Laser OFF" ("Green laser mode")) -> (s? t:f=w1444:enum32{"Laser ON", "Laser OFF", "Interlace"})
      n910 = local read "FPGA error out"() -> (w1450:errorcluster)
      n911 = xnode "Read/Write Control"("FPGA VI Reference In"=w1452, "error in"=w1450, "Invert GI"=w1446, "Invert GI 2"=w1446, "Invert RI"=w1446, "Invert RI 2"=w1446, "Operating Mode"=w1444, "Operating Mode 2"=w1444, "Red Laser Operating Mode"=w1444, "RI Operating Mode 2"=w1444, "P3"=w1476, "I3"=w1477, "D3"=w1478, "Green FB Setpoint"=w1462, "Green FB On/Off"="Green FB On/Off", "Current Out"=w1459, "Green int current ON count adj"="Green int current ON count adj", "Trap Pos FB Monitor T1 or T2"=w1463, "Trap Pos FB Negate Action"=w1464, "Trap Pos. FB Offset Factor"=w1465, "Trap Pos. FB Mult Factor"=w1466, "Force feedback"=FALSE, "AI1 X Scale"=w1468, "Trap Pos to FIFO"=TRUE, "Trap Pos FB Int Count"=w1470, "TTrig Negate Pos"=w1471, "FB Trig Integrate"="FB Trig Integrate", "Diff FB Measurement?"=w1473, "Negate Diff?"="Negate Diff?", "Trap pos. FB Range"=w1447, "Trap Pos. FB Gains"=w1448, "Red FB Setpoint"=w1482, "RI Current Out"=w1486, "P4"=w1488, "I4"=w1489, "D4"=w1490, "Red FB On/Off"="Red FB On/Off", "Dynamic Force FB (Ronen)"=w1449, "RF synth green feedback max"="RF synth green feedback max") -> ("error out"=w1451:errorcluster)  [unwired: 1 out]
      n912 = local write "FPGA error out"(w1451) -> ()
    }
    frame #3 {
      # "Initialize more settings. Should stop using event loops to initialize."
      # "What are these?"
      n913 = local write "Offset (nm)"(0.0 ("Offset (nm)")) -> ()
      n914 = local write "Bead Mean (nm)"(0.0 ("Bead Mean (nm)")) -> ()
      n915 = stacked-sequence {
        frame #0 {
          w1494 = T49."empty" ("mode")
          # "Clear external fluorescence triggering FIFO"
          # "APD loop counts"
          # "Fluorescence loop counts (rates)"
          n916 = local read "APD Integration Time (s)"() -> (w1496:dbl)
          n917 = local read "Interlace ON count"() -> (w1497:u16)
          n918 = call "Smart Buffer (DBL) 1.vi"("mode"=w1494) -> ()  [unwired: 5 in, 6 out]
          n919 = call "Smart Buffer (DBL) 2.vi"("mode"=w1494) -> ()  [unwired: 5 in, 6 out]
          n920 = property on="APD Integration Time (s)" class="DigNum (strict)"("Val(Sgnl)"=w1496) -> ()  [unwired: 2 in, 2 out]
          n921 = property on="Interlace ON count" class="DigNum (strict)"("Val(Sgnl)"=w1497) -> ()  [unwired: 2 in, 2 out]
          "Number of APDs" <- 3.0 ("Number of APDs")
        }
        frame #1 {
          # "Number of APDs affects\nAPD DMA transfer"
          # "General settings for all lasers:"
          # "And includes all laser\nON/OFF settings"
          # "Fluorescent lasers settings:"
          # "Blue laser settings:"
          n922 = local read "Laser interlacing mode"() -> (w1499:enum32{"Laser ON", "Laser OFF", "Interlace"})
          n923 = local read "Invert laser interlacing"() -> (w1498:bool)
          n924 = local read "Blue FB On/Off"() -> (w1500:bool)
          n925 = property on="Blue FB On/Off" class="Bool (strict)"("Val(Sgnl)"=w1500) -> ()  [unwired: 2 in, 2 out]
          n926 = property on="Invert laser interlacing" class="Bool (strict)"("Val(Sgnl)"=w1498) -> ()  [unwired: 2 in, 2 out]
          n927 = property on="Laser interlacing mode" class="RadioBtnsControl (strict)"("Val(Sgnl)"=w1499) -> ()  [unwired: 2 in, 2 out]
        }
        frame #2 {
          w1501 = path "C:/Home/Bustamante Lab/Comstock-LabView-Link.udl" ("connection information")
          # "Database link changed by Ronen - not clear if it matter for the program."
          # "Initialize the database connection"
          n928 = disable-structure shown="Disabled" {
            disable-tunnel: [w1504 _] -> w1502
            disable-tunnel: w1501 -> [w1503 _]
            frame Disabled {
              n929 = call-poly <vilib>:"DB Tools Open Connection.vi"("connection information"=w1503) -> ("connection reference"=w1504:T27)  [unwired: 7 in, 1 out]